vi "Fgen Arb Tester (SS-OCT)_Bscan.vi"() -> ()   [LabVIEW 2012]
doc: "This example shows how to use the Arbitrary Waveform mode to generate on two channels."
uses:
  <instrlib>/niFgen/niFgen.llb/niFgen Output Mode.ctl
  <instrlib>/niFgen/niFgen.llb/niFgen Write Named Waveform (DBL).vi
panel:
  out "Number of A-Scans":i32=500
  in  "File Read Length":i32=-1
  in  "B-Scan":T1={"Active Record Length"=2000, "Duty Cyle Factor"=0.4}
  in  "OCT Signal Data Folder":path=path "C:/Program Files (x86)/National Instruments/LabVIEW 2012/user.lib/Fast OCT/Debug/Arbs/Data/Finger Data"
  in  "CH1 Gain":dbl(knob)=0.5 caption="CH 1 Gain" step=0.0001 scale=0.0..2.5 scale format="%#.7f"
  out "OCT Signals":dbl[][](graph) caption="Graph"
  in  "CH0 Gain":dbl(knob)=0.5 caption="CH 0 Gain" step=0.0001 scale=0.0..2.5 scale format="%#.7f"
  in  "Sample Rate":dbl=250000000.0 format="%.2p"
  in  "stop":bool
  in  "Update":bool
  in  "Sample Clock Source":string(combo)="OnboardClock"
  in  "Resource Name":refnum<k15>="PXI1Slot5"
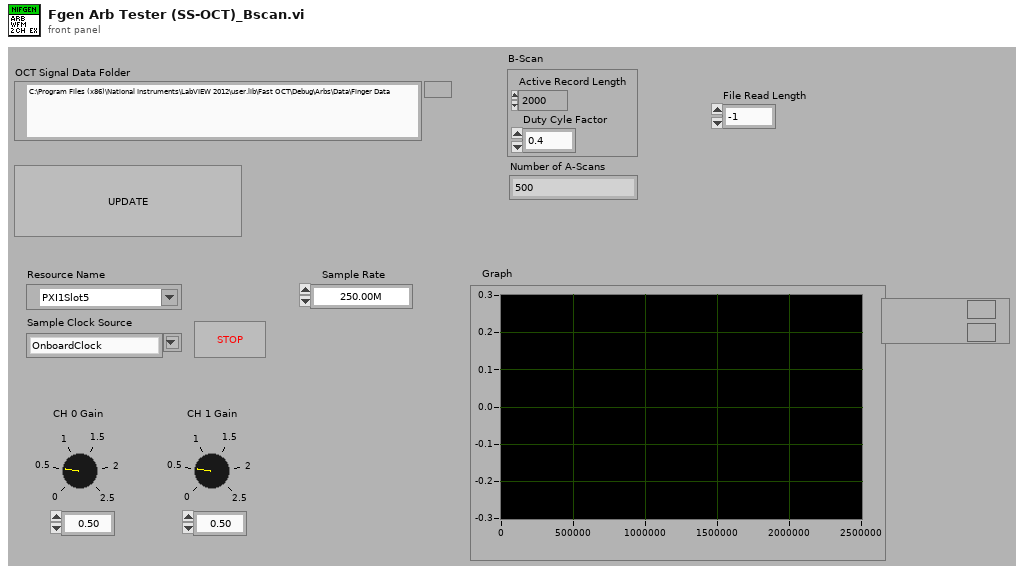
[diagram p1: front panel]
types:
  T1 = cluster{"Active Record Length":i32, "Duty Cyle Factor":dbl}
  T2 = typedef "niFgen Output Mode.ctl" = u32
  T3 = cluster{"Recreated Wfm Size":i32, "Initial Waveform Size":i32, "Number of A-Scans":i32}
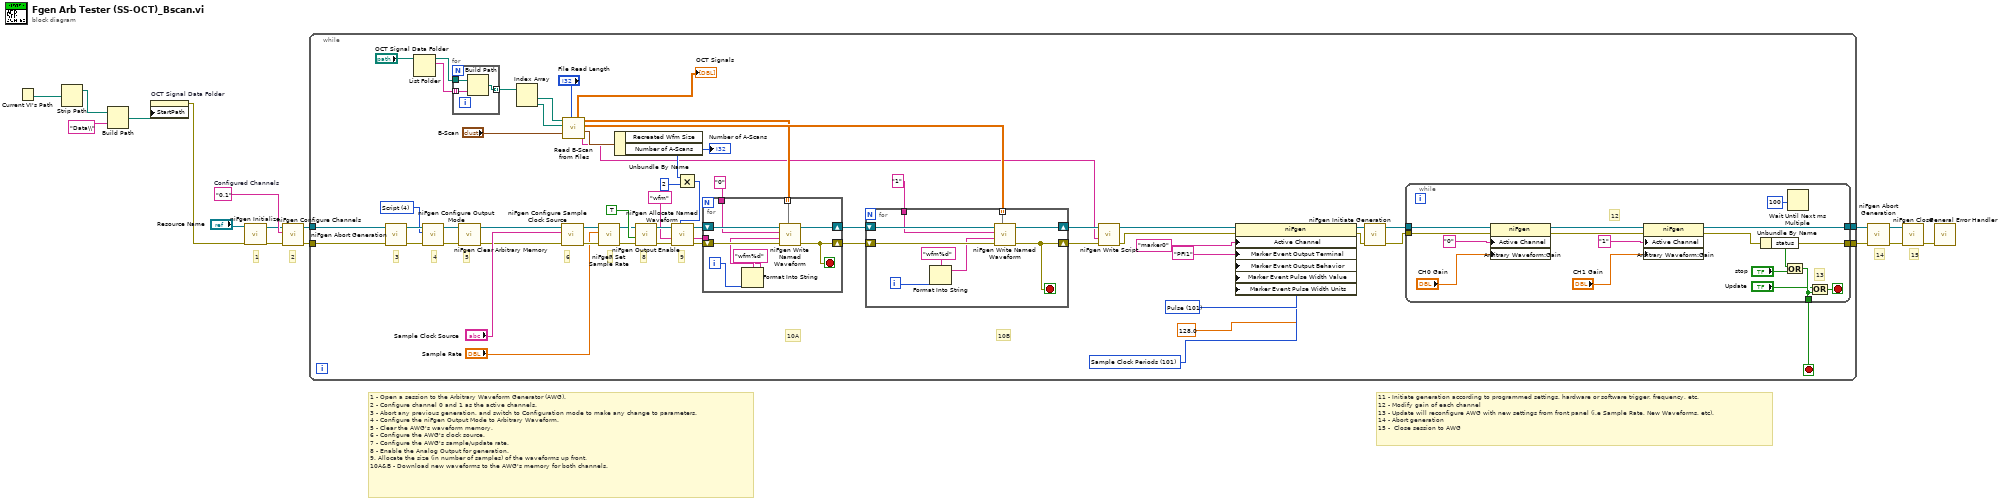
[diagram p0: block diagram]
diagram:
  w10 = "0,1"  # Configured Channels
  # "15"
  # "11 - Initiate generation according to programmed settings, hardware or software trigger, frequency, etc.\n12 - Modify gain of each channel \n13 - Update will reconfigure AWG with new settings from front panel (i.e Sample Rate, New Waveforms, etc).\n14 - Abort generation\n15 -  Close session to AWG"
  # "2"
  # "14"
  # "1"
  # "1 - Open a session to the Arbitrary Waveform Generator (AWG).\n2 - Configure channel 0 and 1 as the active channels.\n3 - Abort any previous generation, and switch to Configuration mode to make any change to parameters.\n4 - Configure the niFgen Output Mode to Arbitrary Waveform.\n5 - Clear the AWG's waveform memory.\n6 - Configure the AWG's clock source.\n7 - Configure the AWG's sample/update rate.\n8 - Enable the Analog Output for generation.\n9. Allocate the size (in number of samples) of the waveforms up front.\n10A&B - Download new waveforms to the AWG's memory for both channels."
  n1 = Current VI's Path() -> (path=w2:path)
  n2 = Strip Path(path=w2) -> (stripped path=w1:path)  [unwired: 1 out]
  n3 = Build Path(base path=w1, name or relative path="Data\\") -> (appended path=w4:path)
  n4 = property on="OCT Signal Data Folder" class="Path"("StartPath"=w4) -> (error out=w5:errorcluster)  [unwired: 2 in, 1 out]
  n5 = call <instrlib>:"niFgen Initialize.vi"("error in (no error)"=w5, "Resource Name"="Resource Name") -> ("error out"=w9:errorcluster, "Instrument Handle Out"=w6:refnum<k15>)  [unwired: 2 in, 6 out]
  n6 = call <instrlib>:"niFgen Configure Channels.vi"("error in (no error)"=w9, "Channels"=w10, "Instrument Handle"=w6) -> ("error out"=w8:errorcluster, "Instrument Handle Out"=w7:refnum<k15>)  [unwired: 7 out]
  n7 = while {
    tunnel: [w62] -> w15
    tunnel: [w74] -> w16
    tunnel: w8 -> [w64]
    tunnel: w7 -> [w73]
    stop <- w75 stop-if-true
    w43 = 101 items=["Sample Clock Periods"=101, "Seconds"=102] ("Events:Marker:Pulse:Width Units")
    w44 = 101 items=["Pulse"=101, "Toggle"=103] ("Events:Marker:Output Behavior")
    w70 = T2 4 items=["Standard Function", "Frequency List", "Arbitrary Waveform", "Arbitrary Sequence", "Script"] ("Output Mode")
    # "10B"
    # "8"
    # "7"
    # "6"
    # "10A"
    # "9"
    # "5"
    # "4"
    # "3"
    n8 = call <instrlib>:"niFgen Abort Generation.vi"("error in (no error)"=w64, "Instrument Handle"=w73) -> ("error out"=w72:errorcluster, "Instrument Handle Out"=w71:refnum<k15>)  [unwired: 8 out]
    n9 = List Folder(path="OCT Signal Data Folder") -> (path out=w22:path, filenames=w21:string[])  [unwired: 3 in, 2 out]
    n10 = call <instrlib>:"niFgen Configure Output Mode.vi"("error in (no error)"=w72, "Output Mode (default: 0=Standard Function)"=w70, "Instrument Handle"=w71) -> ("error out"=w68:errorcluster, "Instrument Handle Out"=w69:refnum<k15>)  [unwired: 6 out]
    n11 = for {
      tunnel: w22 -> [w78]
      tunnel: w21 -> [w77] mode=indexing
      tunnel: [w76] -> w20 mode=indexing
      n12 = Build Path(base path=w78, name or relative path=w77) -> (appended path=w76:path)
    }
    n13 = call <instrlib>:"niFgen Clear Arbitrary Memory.vi"("error in (no error)"=w68, "Instrument Handle"=w69) -> ("error out"=w51:errorcluster, "Instrument Handle Out"=w52:refnum<k15>)  [unwired: 8 out]
    n14 = Index Array(array=w20) -> (element #1=w19:path, element #2=w18:path)  [unwired: 2 in]
    n15 = call <instrlib>:"niFgen Configure Sample Clock Source.vi"("error in (no error)"=w51, "Source (Onboard Clock)"="Sample Clock Source", "Instrument Handle"=w52) -> ("error out"=w66:errorcluster, "Instrument Handle Out"=w67:refnum<k15>)  [unwired: 7 out]
    n16 = call <userlib>:"Read B-Scan from Files.vi"("File Read Length"="File Read Length", "B-Scan"="B-Scan", "Reference Signal"=w18, "OCT Signal"=w19) -> ("Script"=w26:string, "Waveform Info"=w28:T3, "K-Clock Signal"=w31:dbl[][], "OCT Signal"=w30:dbl[][], "Signals"=→"OCT Signals":dbl[][])  [unwired: 3 in]
    n17 = call <instrlib>:"niFgen Set Sample Rate.vi"("error in (no error)"=w66, "Sample Rate (Samp/s)"="Sample Rate", "Instrument Handle"=w67) -> ("error out"=w49:errorcluster, "Instrument Handle Out"=w50:refnum<k15>)  [unwired: 7 out]
    n18 = Unbundle By Name(w28) -> ("Recreated Wfm Size"=w27:i32, "Number of A-Scans"=→"Number of A-Scans":i32)
    n19 = call <instrlib>:"niFgen Output Enable.vi"("error in (no error)"=w49, "Output Enable (default: True)"=TRUE ("output enable"), "Instrument Handle"=w50) -> ("error out"=w58:errorcluster, "Instrument Handle Out"=w57:refnum<k15>)  [unwired: 1 in, 6 out]
    n20 = Multiply(x=w27, y=u32 2) -> (x*y=w36:u32)
    n21 = call <instrlib>:"niFgen Allocate Named Waveform.vi"("Waveform Size"=w36, "error in (no error)"=w58, "Waveform Name"="wfm" ("Channel Name"), "Instrument Handle"=w57) -> ("error out"=w56:errorcluster, "Waveform Name Out"=w40:string, "Instrument Handle Out"=w55:refnum<k15>)  [unwired: 5 in]
    n22 = for {
      tunnel: "0" ("Channel Name") -> [w84]
      tunnel: w40 -> [_]
      tunnel: w30 -> [w83] mode=indexing
      shift-right: [w82] -> w60
      shift-left: w56 -> [w86]
      shift-right: [w87] -> w59
      shift-left: w55 -> [w85]
      i -> [w80]
      stop <- w82 stop-if-true
      n23 = Format Into String(format string="wfm%d", w80) -> (resulting string=w79:string)  [unwired: 2 in, 1 out]
      n24 = call-poly <instrlib>:"niFgen Write Named Waveform.vi"("Waveform Data"=w83, "error in (no error)"=w86, "Waveform Name"=w79, "Channel Name"=w84, "Instrument Handle"=w85) -> ("error out"=w82:errorcluster, "Instrument Handle Out"=w87:refnum<k15>)  [unwired: 4 in, 1 out]
    }
    n25 = for {
      tunnel: "1" ("Channel Name") -> [w94]
      tunnel: w31 -> [w93] mode=indexing
      shift-right: [w92] -> w33
      shift-left: w59 -> [w95]
      shift-right: [w88] -> w32
      shift-left: w60 -> [w96]
      i -> [w91]
      stop <- w88 stop-if-true
      n26 = Format Into String(format string="wfm%d", w91) -> (resulting string=w90:string)  [unwired: 2 in, 1 out]
      n27 = call-poly <instrlib>:"niFgen Write Named Waveform.vi"("Waveform Data"=w93, "error in (no error)"=w96, "Waveform Name"=w90, "Channel Name"=w94, "Instrument Handle"=w95) -> ("error out"=w88:errorcluster, "Instrument Handle Out"=w92:refnum<k15>)  [unwired: 4 in, 1 out]
    }
    n28 = call <instrlib>:"niFgen Write Script.vi"("error in (no error)"=w32, "Script"=w26, "Instrument Handle"=w33) -> ("error out"=w38:errorcluster, "Instrument Handle Out"=w39:refnum<k15>)  [unwired: 7 in]
    n29 = property class="niFgen"(reference=w39, error in=w38, "Active Channel"="marker0", "Marker Event Output Terminal"="PFI1" ("Events:Marker:Output Terminal"), "Marker Event Output Behavior"=w44, "Marker Event Pulse Width Value"=128.0 ("Events:Marker:Pulse:Width Value"), "Marker Event Pulse Width Units"=w43) -> (reference out=w46:refnum<k15>, error out=w45:errorcluster)
    n30 = call <instrlib>:"niFgen Initiate Generation.vi"("error in (no error)"=w45, "Instrument Handle"=w46) -> ("error out"=w47:errorcluster, "Instrument Handle Out"=w48:refnum<k15>)  [unwired: 8 out]
    n31 = while {
      tunnel: [w97] -> w74
      tunnel: w48 -> [w106]
      tunnel: [w108] -> w75
      tunnel: w47 -> [w105]
      tunnel: [w98] -> w62
      stop <- w111 stop-if-true
      # "12"
      # "13"
      n32 = property class="niFgen"(reference=w106, error in=w105, "Active Channel"="0", "Arbitrary Waveform:Gain"="CH0 Gain") -> (reference out=w102:refnum<k15>, error out=w101:errorcluster)
      n33 = property class="niFgen"(reference=w102, error in=w101, "Active Channel"="1", "Arbitrary Waveform:Gain"="CH1 Gain") -> (reference out=w97:refnum<k15>, error out=w98:errorcluster)
      n34 = Unbundle By Name(w98) -> ("status"=w109:bool)
      n35 = Or(x=w109, y="stop") -> (x .or. y?=w108:bool)
      n36 = Wait Until Next ms Multiple(millisecond multiple=u32 100) -> ()  [unwired: 1 out]
      n37 = Or(x="Update", y=w108) -> (x .or. y?=w111:bool)
    }
  }
  n38 = call <instrlib>:"niFgen Abort Generation.vi"("error in (no error)"=w15, "Instrument Handle"=w16) -> ("error out"=w14:errorcluster, "Instrument Handle Out"=w13:refnum<k15>)  [unwired: 8 out]
  n39 = call <instrlib>:"niFgen Close.vi"("error in (no error)"=w14, "Instrument Handle"=w13) -> ("error out"=w11:errorcluster)  [unwired: 9 out]
  n40 = call <vilib>:"General Error Handler.vi"("error in (no error)"=w11) -> ()  [unwired: 1 in, 14 out]
